vi "ScanDelay_FTIR_BBnorm.vi"() -> ()   [LabVIEW 2022 SP3] (continued)
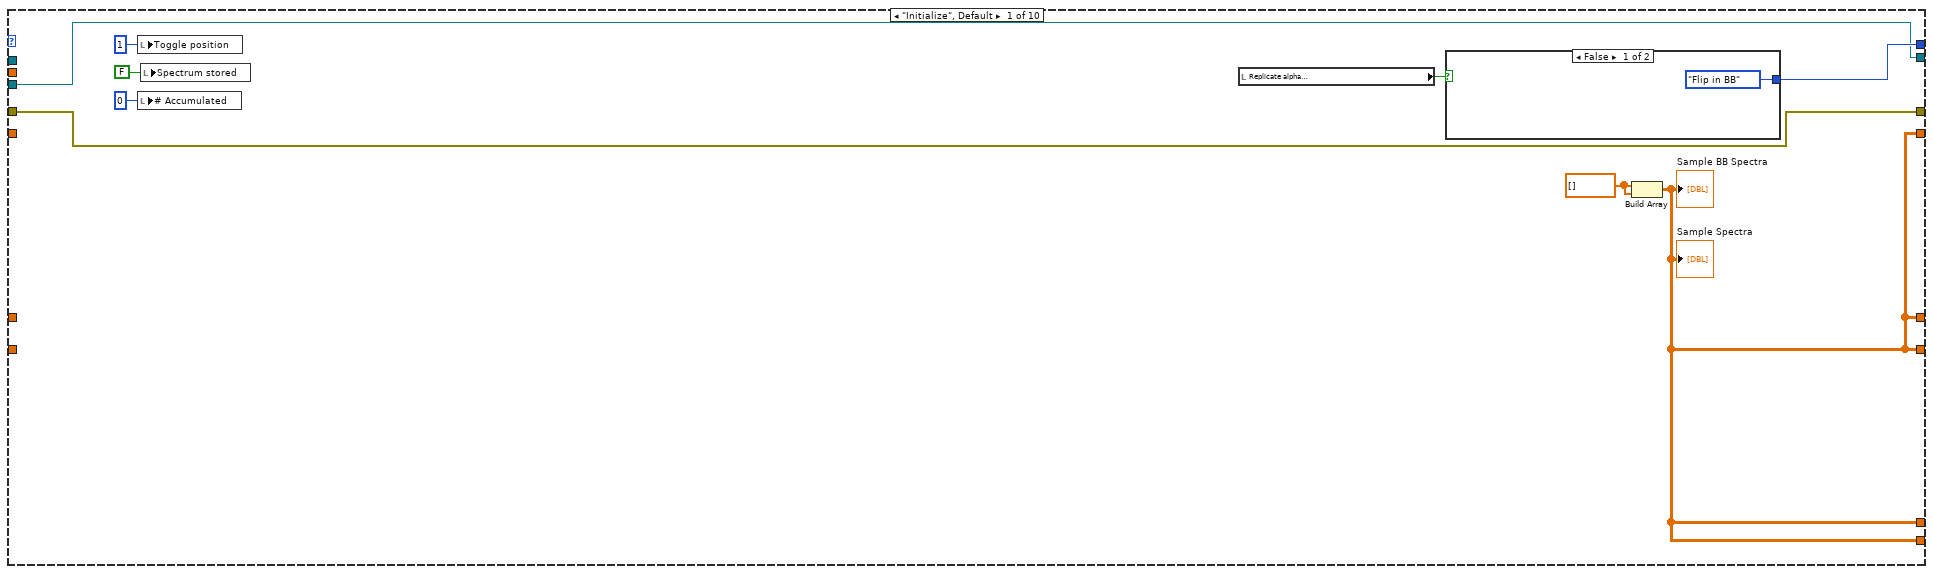
[diagram p2: hidden frame]
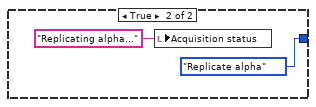
[diagram p3: hidden frame]
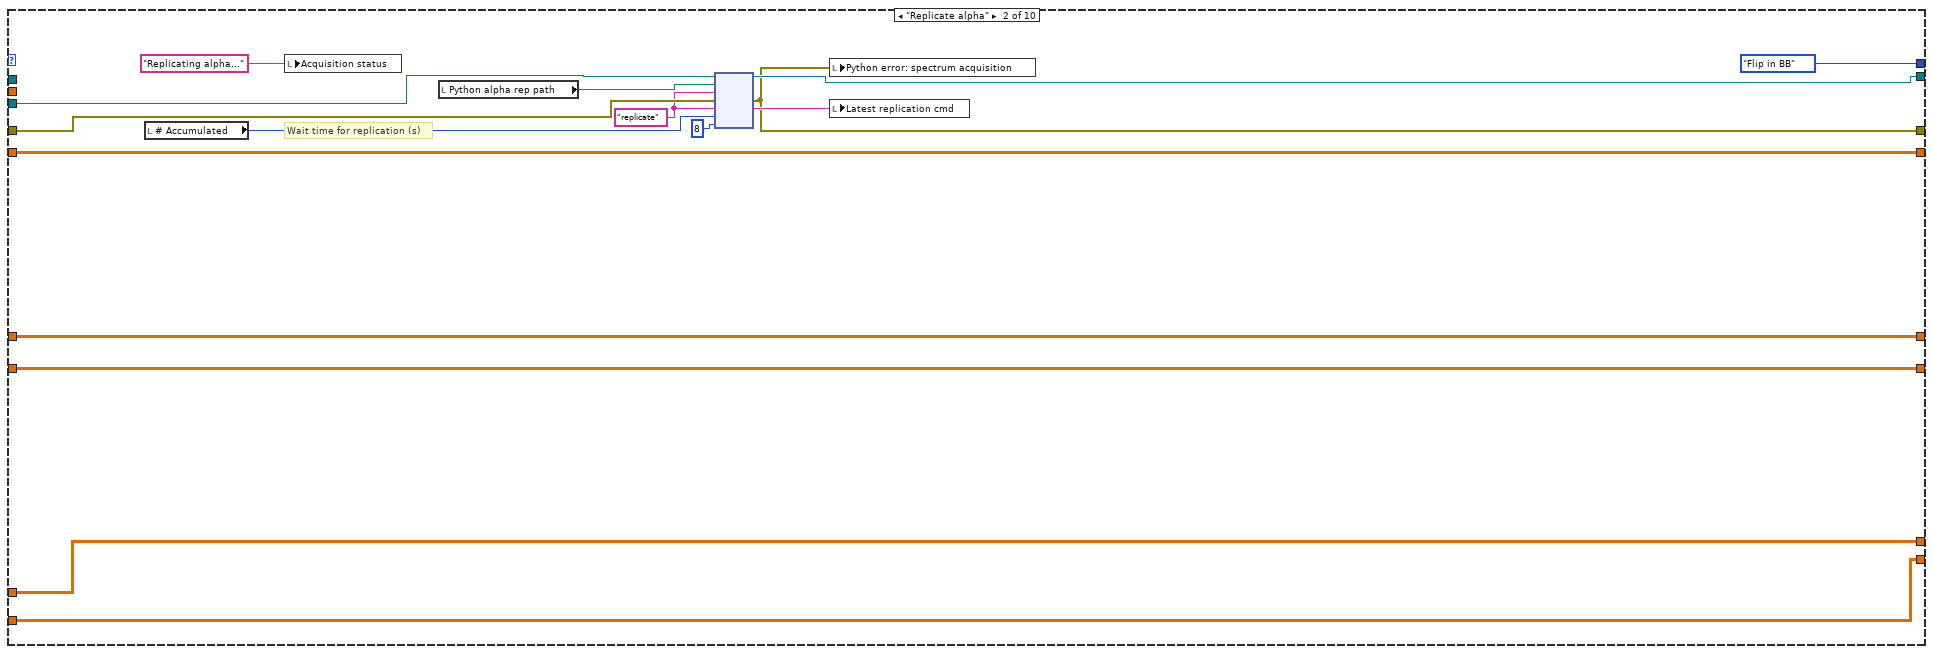
[diagram p4: hidden frame]
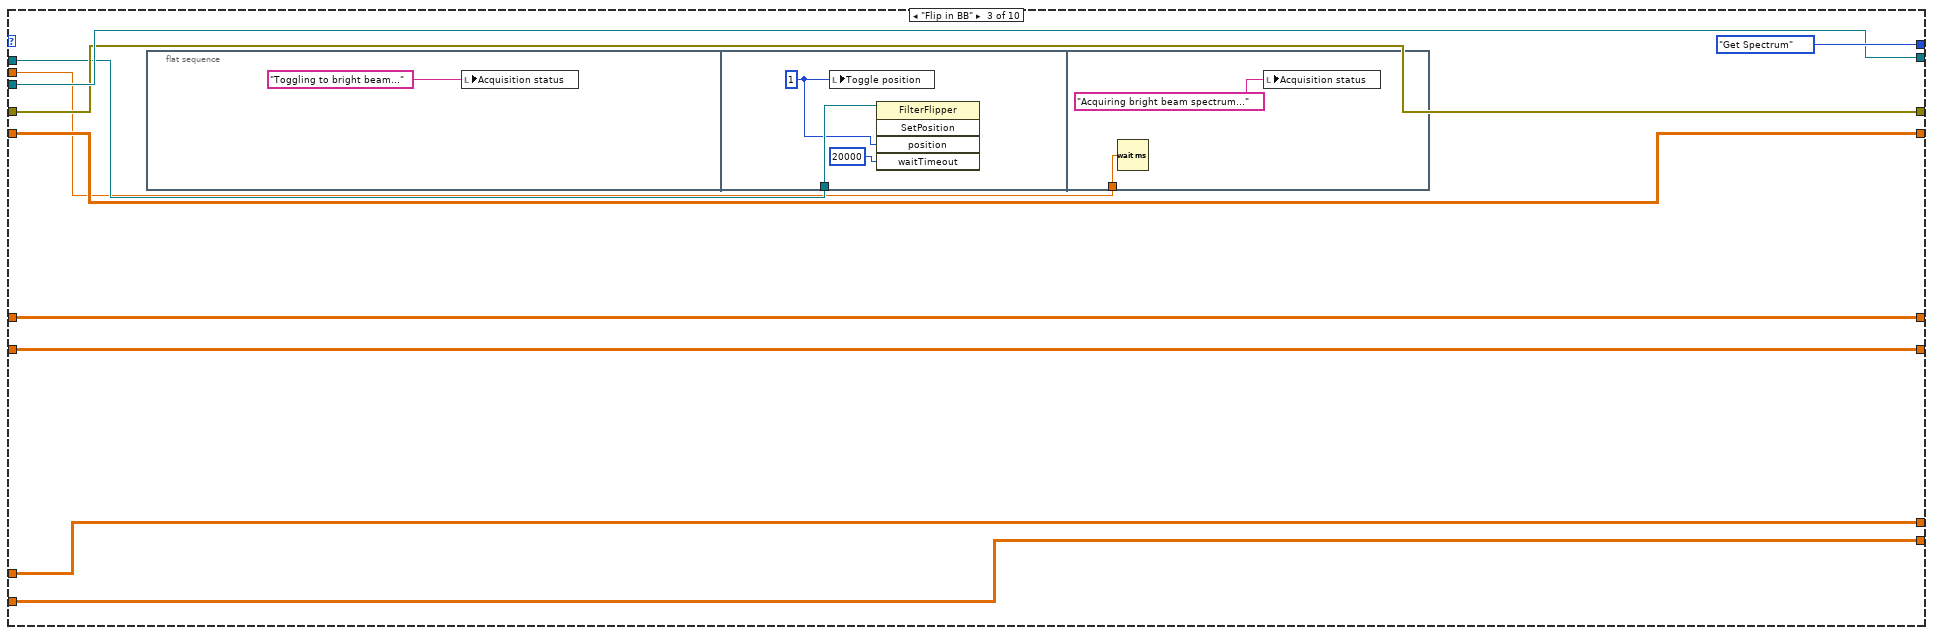
[diagram p5: hidden frame]
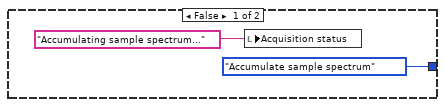
[diagram p6: hidden frame]
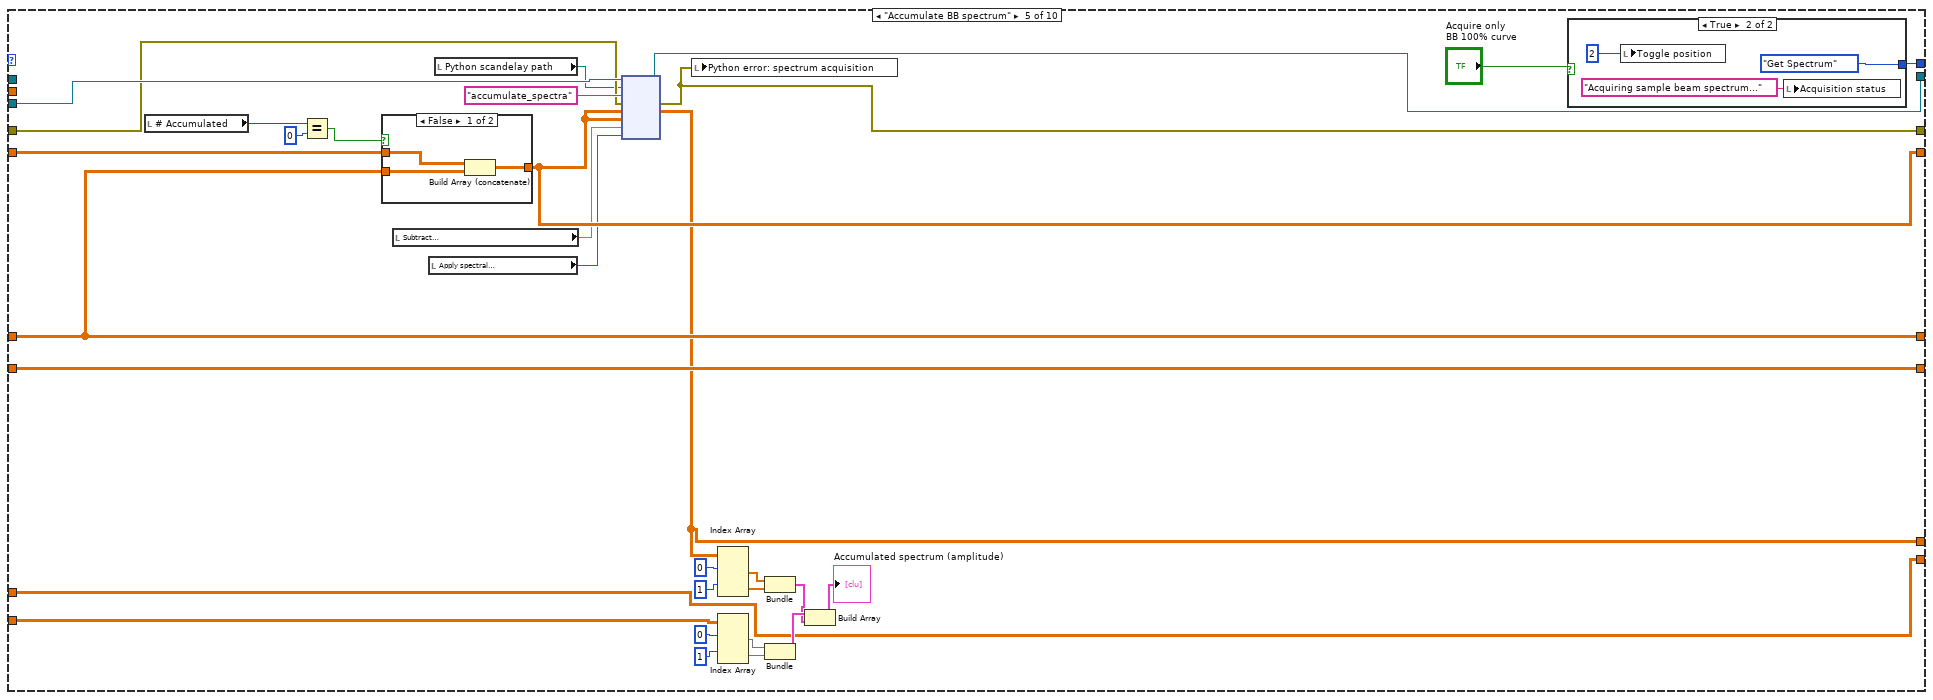
[diagram p7: hidden frame]
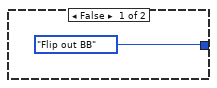
[diagram p8: hidden frame]
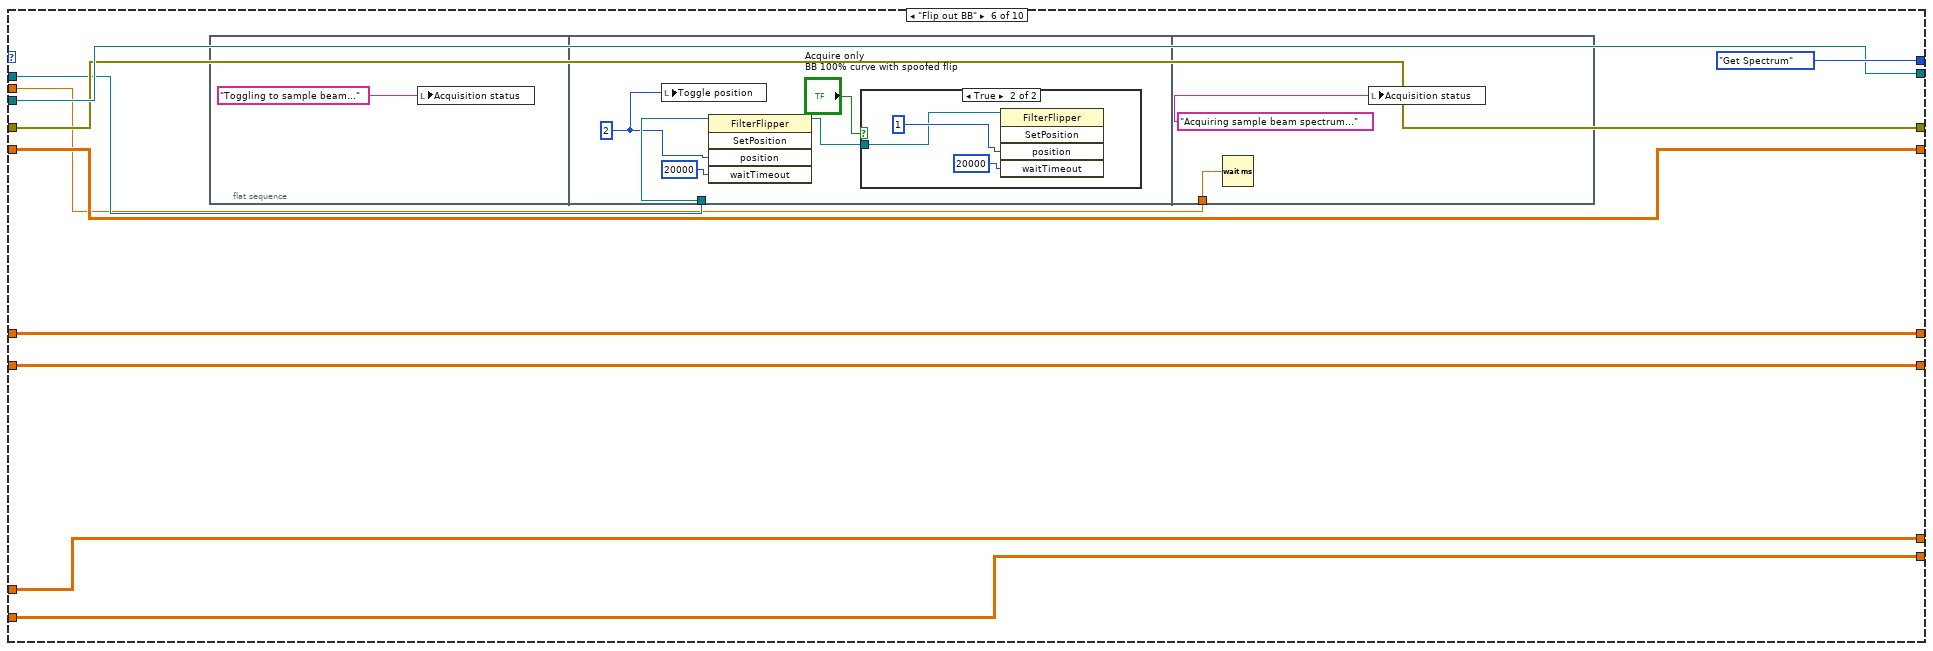
[diagram p10: hidden frame]
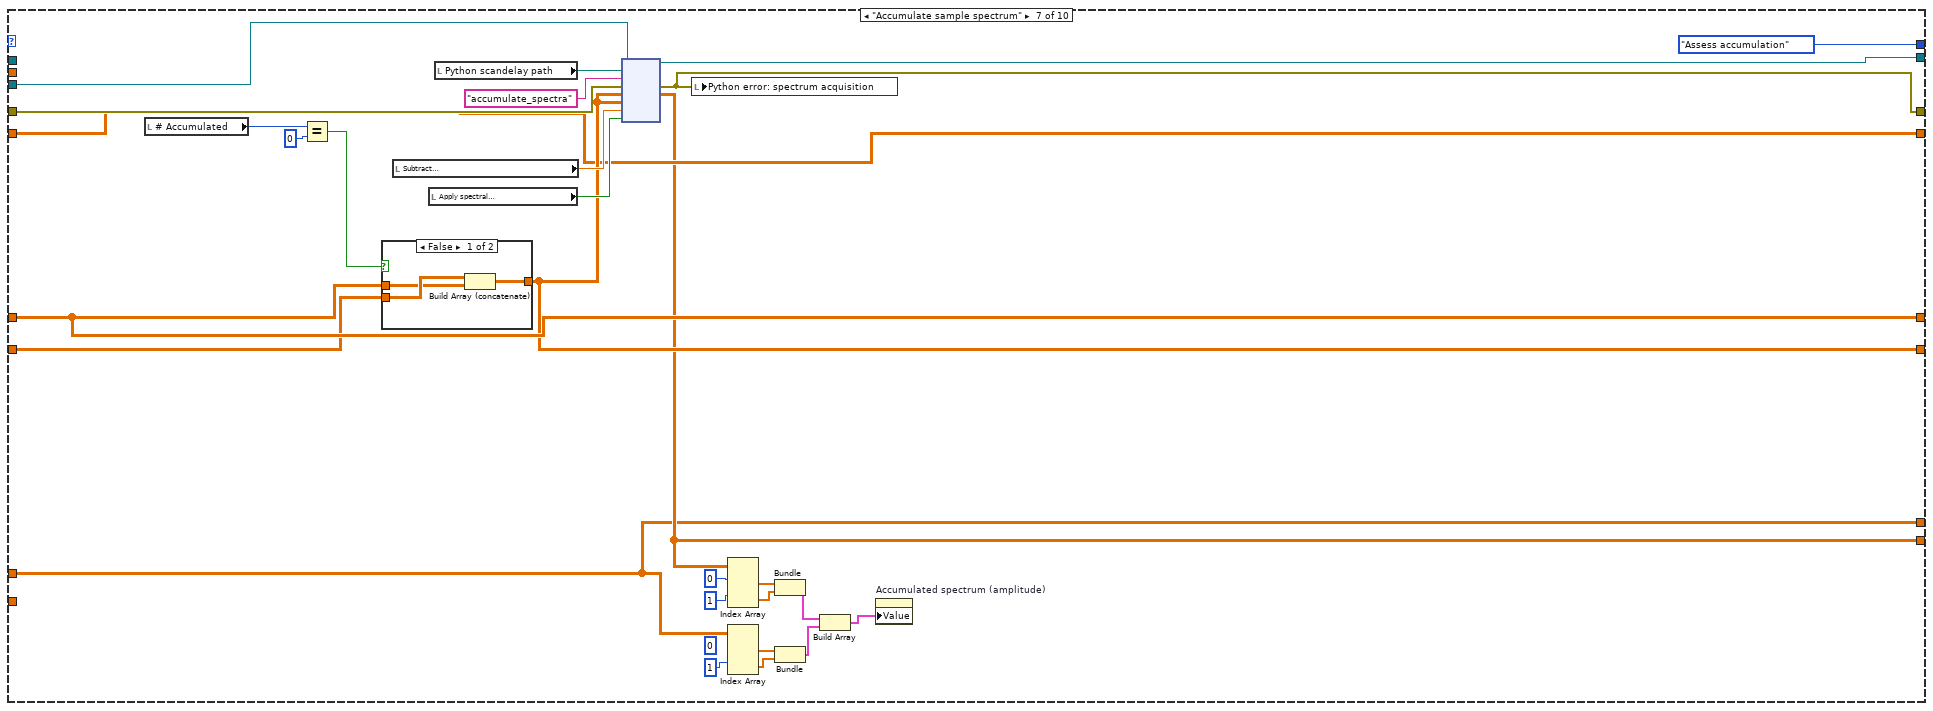
[diagram p12: hidden frame]
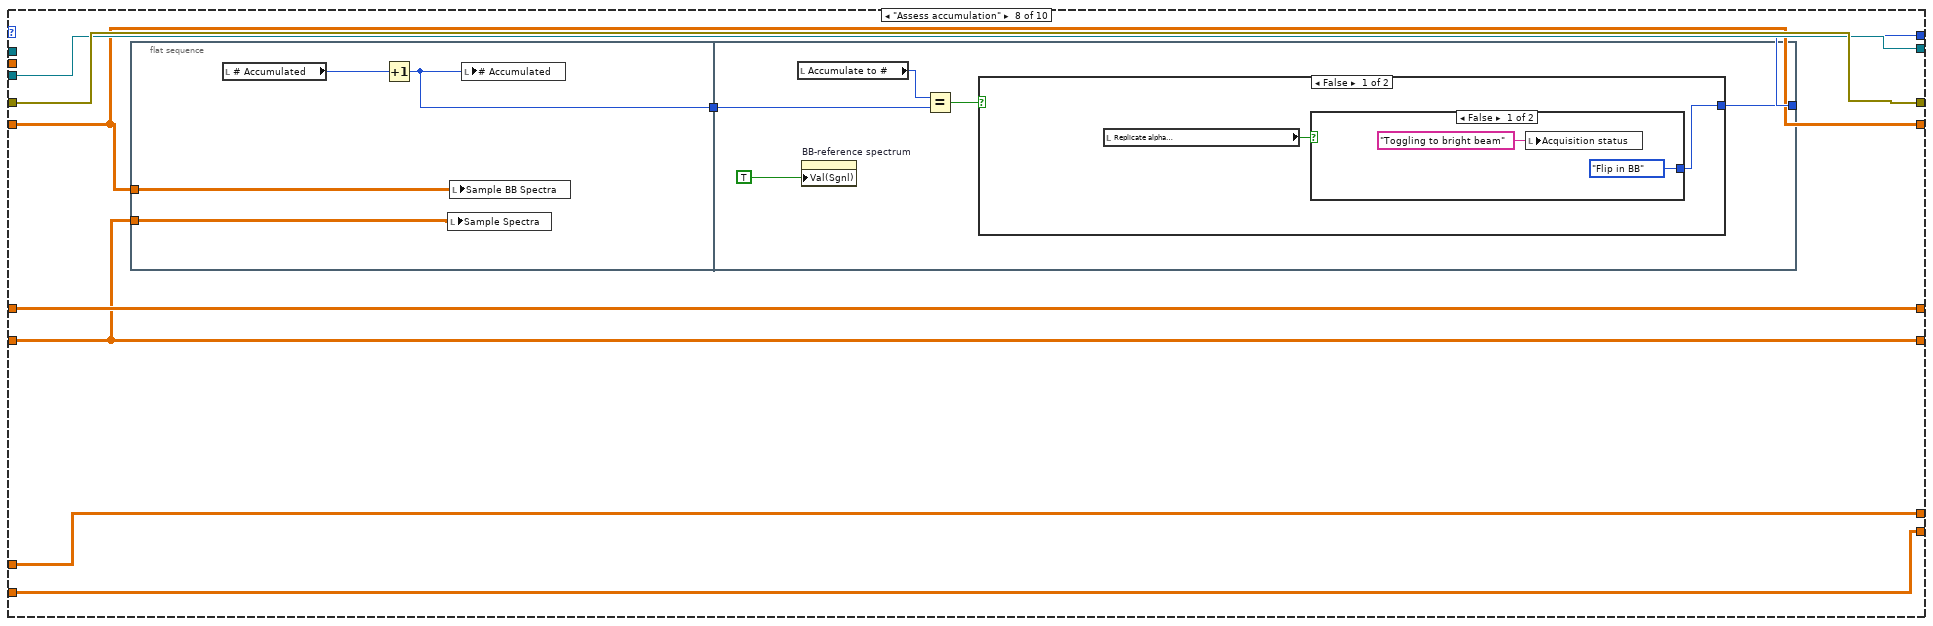
[diagram p14: hidden frame]
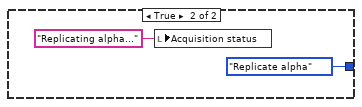
[diagram p15: hidden frame]
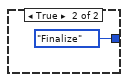
[diagram p16: hidden frame]
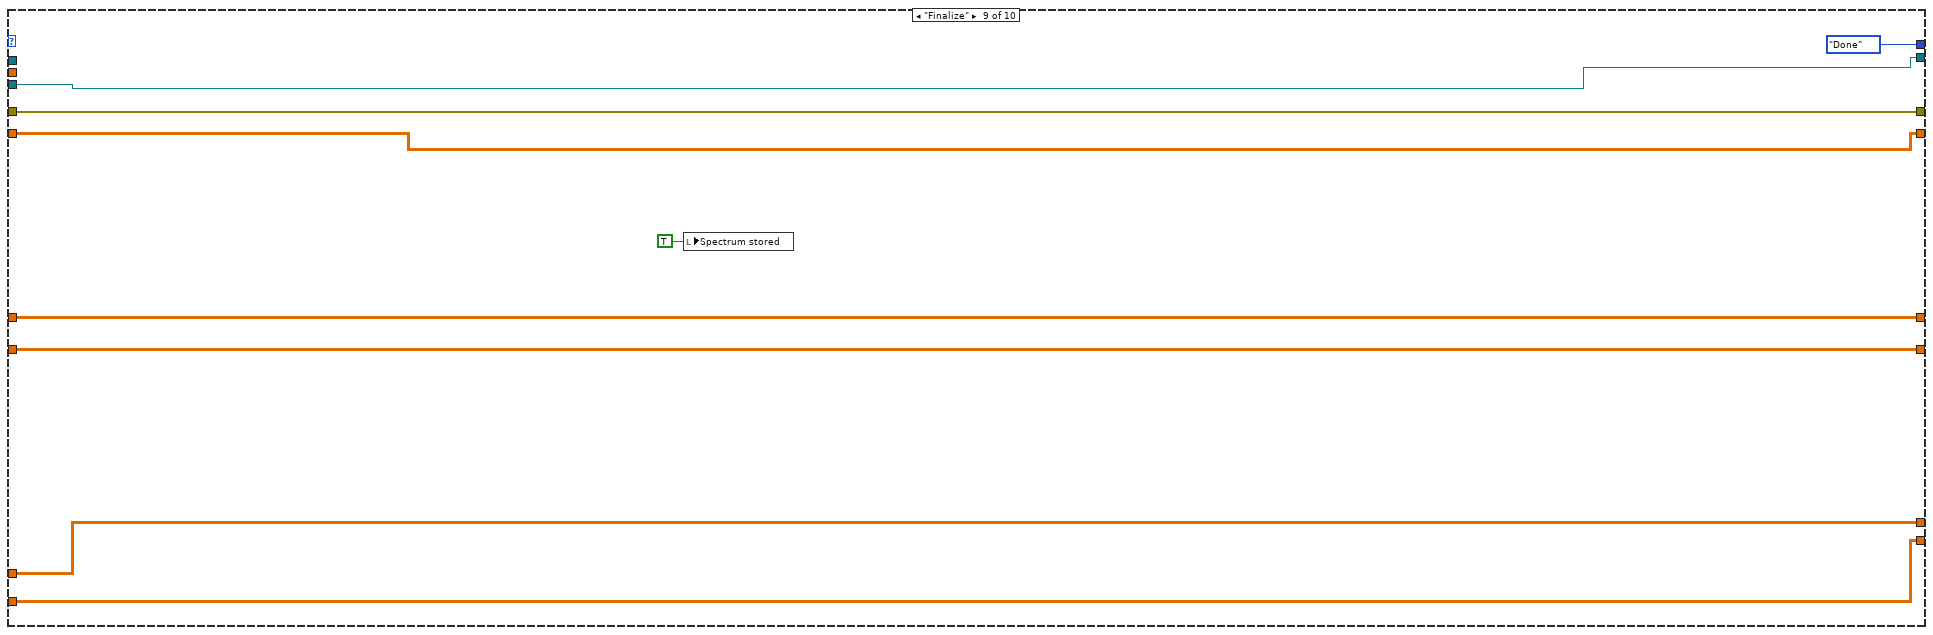
[diagram p17: hidden frame]
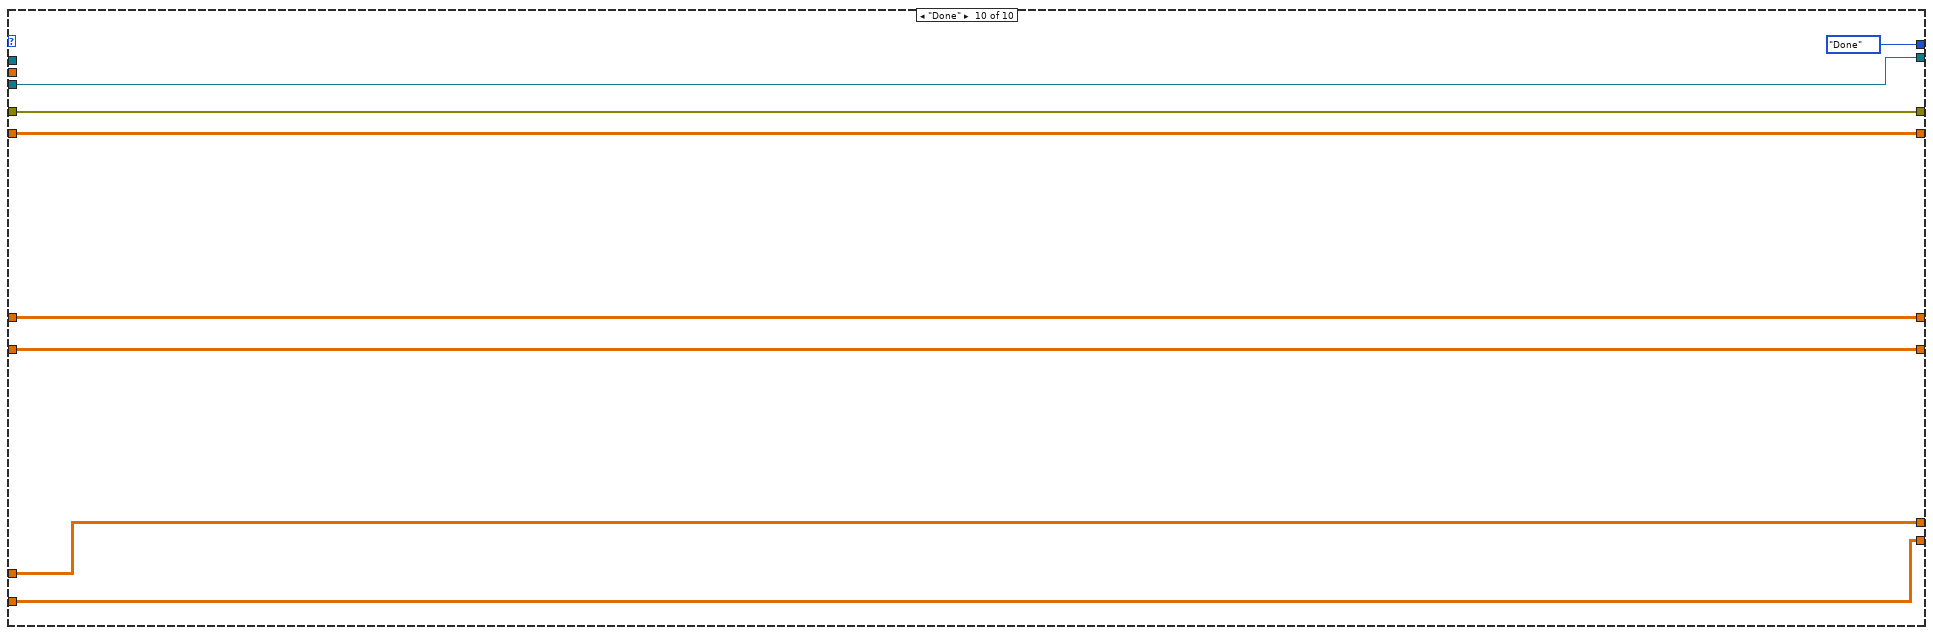
[diagram p18: hidden frame]
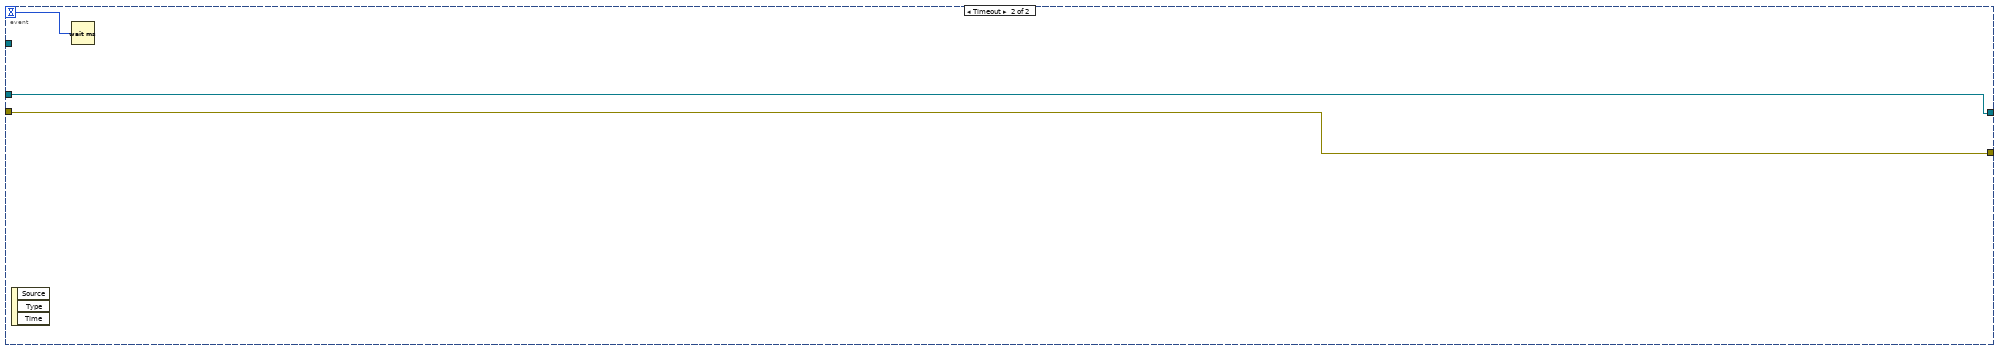
[diagram p19: hidden frame]
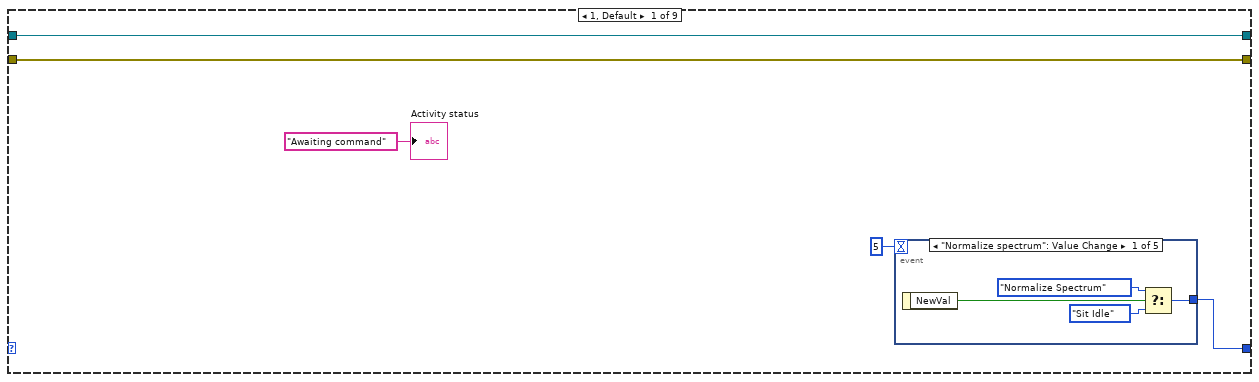
[diagram p20: hidden frame]
              n117 = Equal?(x=w324, y=0) -> (x = y?=w322:bool)
              n118 = case shown="False" w322 {
                tunnel: w310 -> [w331 w333]
                tunnel: w325 -> [w332 _]
                tunnel: [w330 w333] -> w316
                frame False {
                  n119 = Build Array (concatenate)(w332, w331) -> (w330:dbl[][])
                }
                frame True {
                }
              }
              n120 = local read "Subtract\nphase slope\n (2pi * dx)"() -> (w308:dbl)
              n121 = local read "Apply spectral\nenvelope"() -> (w315:bool)
              n122 = local read "Python scandelay path"() -> (w317:path)
              n123 = node(w320, w317, "accumulate_spectra", w319, w316, w316, w308, w315) -> (w318:refnum<k35>, w307:errorcluster, w297:dbl[][])  [unwired: 3 in, 2 out]
              n124 = local write "Python error: spectrum acquisition"(w307) -> ()
              n125 = Index Array(array=w297, index (row) #1=0, index (row) #2=1) -> (element #1=w312:dbl[], element #2=w311:dbl[])  [unwired: 2 in]
              n126 = Index Array(array=w296, index (row) #1=0, index (row) #2=1) -> (element #1=w303:dbl[], element #2=w302:dbl[])  [unwired: 2 in]
              n127 = Bundle("Output spectrum"=w312, "Output spectrum"=w311) -> (w299:T1)  [unwired: 1 in]
              n128 = Bundle("Output spectrum"=w303, "Output spectrum"=w302) -> (w300:T1)  [unwired: 1 in]
              n129 = Build Array(w300, w299) -> (→"Accumulated spectrum (amplitude)":T2)
              n130 = case shown="True" "Acquire only\nBB 100% curve" {
                tunnel: [Control_GetSpectrum_BBnorm."Flip out BB" Control_GetSpectrum_BBnorm."Get Spectrum"] -> w309
                frame False {
                }
                frame True {
                  n131 = local write "Toggle position"(2) -> ()
                  n132 = local write "Acquisition status"("Acquiring sample beam spectrum...") -> ()
                }
              }
            }
            frame "Flip out BB" {
              n133 = flat-sequence {
                tunnel: w337 -> [w349]
                tunnel: w336 -> [w353]
                frame #0 {
                  n134 = local write "Acquisition status"("Toggling to sample beam...") -> ()
                }
                frame #1 {
                  w347 = 2
                  n135 = local write "Toggle position"(w347) -> ()
                  n136 = invoke class="FilterFlipper" method="SetPosition"(reference=w349, "position"=w347, "waitTimeout"=20000) -> (reference out=w345:refnum<k24>)  [unwired: 2 in, 4 out]
                  n137 = case shown="True" "Acquire only\nBB 100% curve with spoofed flip" {
                    tunnel: w345 -> [_ w350]
                    frame False {
                    }
                    frame True {
                      n138 = invoke class="FilterFlipper" method="SetPosition"(reference=w350, "position"=1, "waitTimeout"=20000) -> ()  [unwired: 2 in, 5 out]
                    }
                  }
                }
                frame #2 {
                  n139 = Wait (ms)(milliseconds to wait=w353) -> ()  [unwired: 1 out]
                  n140 = local write "Acquisition status"("Acquiring sample beam spectrum...") -> ()
                }
              }
            }
            frame "Accumulate sample spectrum" {
              (unwired) 0
              n141 = local read "# Accumulated"() -> (w382:i32)
              n142 = Equal?(x=w382, y=0) -> (x = y?=w380:bool)
              n143 = case shown="False" w380 {
                tunnel: w369 -> [w384 w386]
                tunnel: w366 -> [w385 _]
                tunnel: [w383 w386] -> w365
                frame False {
                  n144 = Build Array (concatenate)(w385, w384) -> (w383:dbl[][])
                }
                frame True {
                }
              }
              n145 = local read "Subtract\nphase slope\n (2pi * dx)"() -> (w367:dbl)
              n146 = local read "Apply spectral\nenvelope"() -> (w374:bool)
              n147 = local read "Python scandelay path"() -> (w375:path)
              n148 = node(w378, w375, "accumulate_spectra", w377, w365, w365, w367, w374) -> (w376:refnum<k35>, w364:errorcluster, w356:dbl[][])  [unwired: 3 in, 2 out]
              n149 = local write "Python error: spectrum acquisition"(w364) -> ()
              n150 = Index Array(array=w356, index (row) #1=0, index (row) #2=1) -> (element #1=w371:dbl[], element #2=w370:dbl[])  [unwired: 2 in]
              n151 = Index Array(array=w355, index (row) #2=1) -> (element #1=w361:dbl[], element #2=w360:dbl[])  [unwired: 3 in]
              n152 = Bundle("Output spectrum"=w371, "Output spectrum"=w370) -> (w363:T1)  [unwired: 1 in]
              n153 = Bundle("Output spectrum"=w361, "Output spectrum"=w360) -> (w359:T1)  [unwired: 1 in]
              n154 = Build Array(w363, w359) -> (w357:T2)
              n155 = property on="Accumulated spectrum (amplitude)" class="XYGraph (strict)"("Value"=w357) -> ()  [unwired: 2 in, 2 out]
            }
            frame "Assess accumulation" {
              n156 = flat-sequence {
                tunnel: [w398] -> w393
                tunnel: w388 -> [w397]
                tunnel: w387 -> [w396]
                tunnel: w393 -> [w403]
                tunnel: [w401] -> w392
                frame #0 {
                  n157 = local read "# Accumulated"() -> (w399:i32)
                  n158 = Increment(x=w399) -> (x+1=w398:i32)
                  n159 = local write "Sample Spectra"(w396) -> ()
                  n160 = local write "Sample BB Spectra"(w397) -> ()
                  n161 = local write "# Accumulated"(w398) -> ()
                }
                frame #1 {
                  n162 = local read "Accumulate to #"() -> (w404:i32)
                  n163 = property on="BB-reference spectrum" class="Bool (strict)"("Val(Sgnl)"=TRUE) -> ()  [unwired: 2 in, 2 out]
                  n164 = Equal?(x=w404, y=w403) -> (x = y?=w402:bool)
                  n165 = case shown="False" w402 {
                    tunnel: [w405 Control_GetSpectrum_BBnorm."Finalize"] -> w401
                    frame False {
                      n166 = local read "Replicate alpha\non accumulation"() -> (w406:bool)
                      n167 = case shown="False" w406 {
                        tunnel: [Control_GetSpectrum_BBnorm."Flip in BB" Control_GetSpectrum_BBnorm."Replicate alpha"] -> w405
                        frame False {
                          n168 = local write "Acquisition status"("Toggling to bright beam") -> ()
                        }
                        frame True {
                          n169 = local write "Acquisition status"("Replicating alpha...") -> ()
                        }
                      }
                    }
                    frame True {
                    }
                  }
                }
              }
            }
            frame "Finalize" {
              n170 = local write "Spectrum stored"(TRUE) -> ()
            }
            frame "Done" {
            }
          }
          n171 = Or(x=w209, y=w208) -> (x .or. y?=w207:bool)
          n172 = Or(x=w210, y=w207) -> (x .or. y?=w206:bool)
          n173 = Wait (ms)(milliseconds to wait=5) -> ()  [unwired: 1 out]
        }
        n174 = local write "Acquire spectrum"(w191) -> ()
        n175 = local write "Cancel\nacquisition"(w191) -> ()
      }
      event Timeout {
        n176 = event-data() -> ()  [unwired: 1 in, 3 out]
        n177 = Wait (ms)(milliseconds to wait=w431) -> ()  [unwired: 1 out]
      }
    }
    n178 = Wait (ms)(milliseconds to wait=5) -> ()  [unwired: 1 out]
    n179 = local read "Halt program"() -> (w190:bool)
    "Acquisition status" <- "Ready to acquire spectrum"
  }
  n180 = Close Python Session(session in=w17, error in=w16) -> (11:w13:errorcluster)
  n181 = local write "Python error: activity loop"(w13) -> ()
  n182 = Close Python Session(session in=w2, error in=w1) -> ()  [unwired: 1 out]
